vi "Generalized Phase Extraction.vi"(6 "sampling info":cluster{"Fs":dbl, "#s":dbl}={"Fs"=100000000.0, "#s"=1000000.0}, 7 "sampling freq: fs":dbl=80000.0, 8 "dt":dbl=1e-08, 9 "order":i32=2, 10 "low cutoff freq: fl":dbl=10.0, 11 "Input Data":dbl[](array[numeric])=array[1000000 elements]) -> (1 "Squeezing Phase Array":dbl[](graph), 2 "detected phase (deg)":dbl format="%.2p", 3 "detected frequency":dbl format="%.4p", 4 "Normalized Envelope":waveform(dbl)(graph), 5 "Envelope":dbl[](graph))   [LabVIEW 2009]
uses:
  <vilib>/measure/matone.llb/Extract Single Tone Information 1 Chan.vi
  <vilib>/Analysis/3filter.llb/Butterworth Filter (DBL).vi
  <vilib>/Analysis/NI_AALBase.lvlib
  <vilib>/measure/NI_MAPro.lvlib
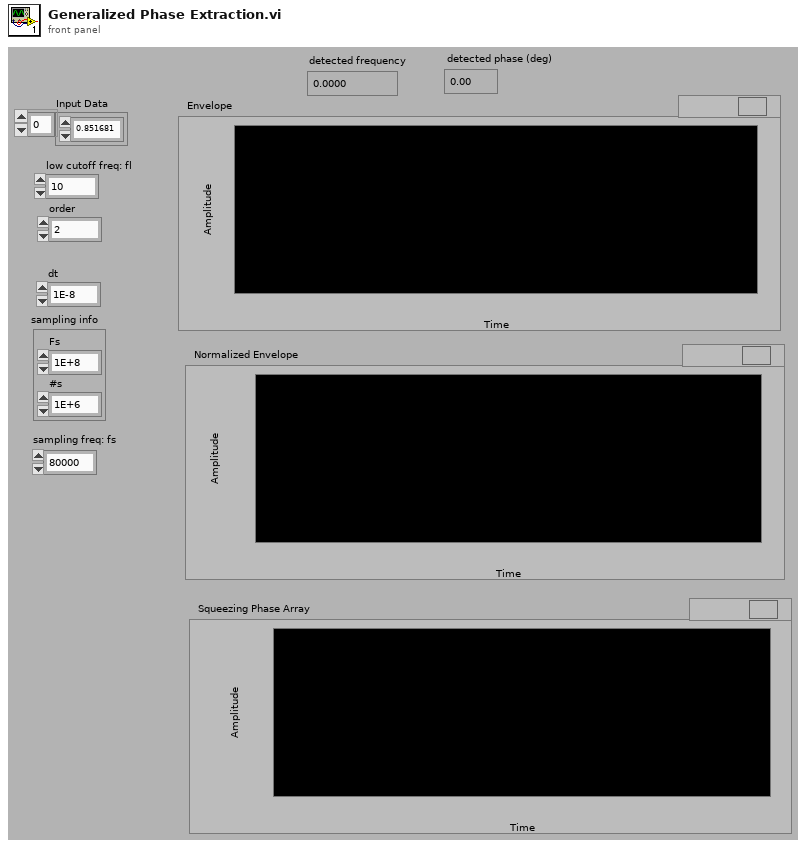
[diagram p1: front panel]
types:
  T1 = enum32{"Lowpass", "Highpass", "Bandpass", "Bandstop"}
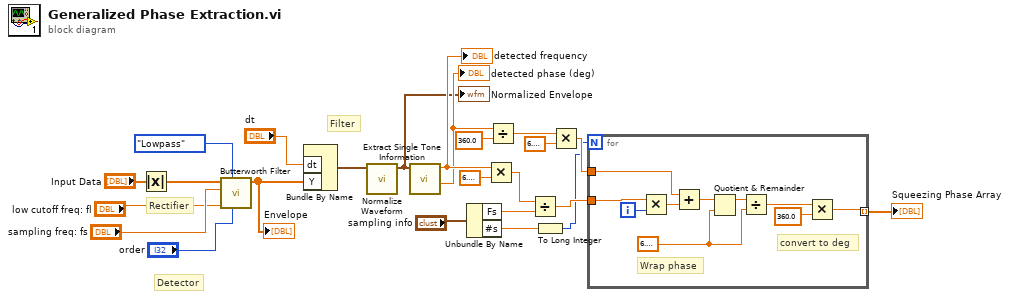
[diagram p0: block diagram]
diagram:
  # "Detector"
  # "Filter"
  # "Rectifier"
  n1 = Absolute Value(x="Input Data") -> (abs(x)=w3:dbl[])
  n2 = call-poly <vilib>:"Butterworth Filter.vi"("order"="order", "filter type"=T1."Lowpass", "low cutoff freq: fl"="low cutoff freq: fl", "sampling freq: fs"="sampling freq: fs", "X"=w3) -> ("Filtered X"=w22:dbl[])  [unwired: 3 in, 1 out]
  "Envelope" <- w22
  n3 = Bundle By Name("dt"="dt", "Y"=w22) -> (w8:waveform(dbl))  [unwired: 1 in]
  n4 = call <vilib>:"Normalize Waveform.vi"("waveform in"=w8) -> ("normalized waveform"=w9:waveform(dbl))  [unwired: 7 in, 3 out]
  "Normalized Envelope" <- w9
  n5 = call-poly <vilib>:"Extract Single Tone Information.vi"("time signal in"=w9) -> ("detected phase (deg)"=w20:dbl, "detected frequency"=w21:dbl)  [unwired: 5 in, 4 out]
  "detected frequency" <- w21
  "detected phase (deg)" <- w20
  n6 = Unbundle By Name("sampling info") -> ("Fs"=w11:dbl, "#s"=w10:dbl)
  n7 = Multiply(x=w21, y=6.283185307179586) -> (x*y=w14:dbl)
  n8 = Divide(x=w20, y=360.0) -> (x/y=w17:dbl)
  n9 = Divide(x=w14, y=w11) -> (x/y=w13:dbl)
  n10 = To Long Integer(number=w10) -> (32bit integer=w1:i32)
  n11 = Multiply(x=w17, y=6.283185307179586) -> (x*y=w12:dbl)
  n12 = for {
    N: w1 -> [_]
    tunnel: w13 -> [w34]
    tunnel: w12 -> [w33]
    tunnel: [w28] -> w24 mode=indexing
    i -> [w25]
    w31 = 6.283185307179586
    # "convert to deg"
    # "Wrap phase"
    n13 = Multiply(x=w34, y=w25) -> (x*y=w32:dbl)
    n14 = Add(x=w33, y=w32) -> (x+y=w27:dbl)
    n15 = Quotient & Remainder(x=w27, y=w31) -> (x-y*floor(x/y)=w26:dbl)  [unwired: 1 out]
    n16 = Divide(x=w26, y=w31) -> (x/y=w30:dbl)
    n17 = Multiply(x=w30, y=360.0) -> (x*y=w28:dbl)
  }
  "Squeezing Phase Array" <- w24
